vi "Velociprobe_Nanopositioner_Control_RT 3.vi"() -> ()   [LabVIEW 2015] (continued)
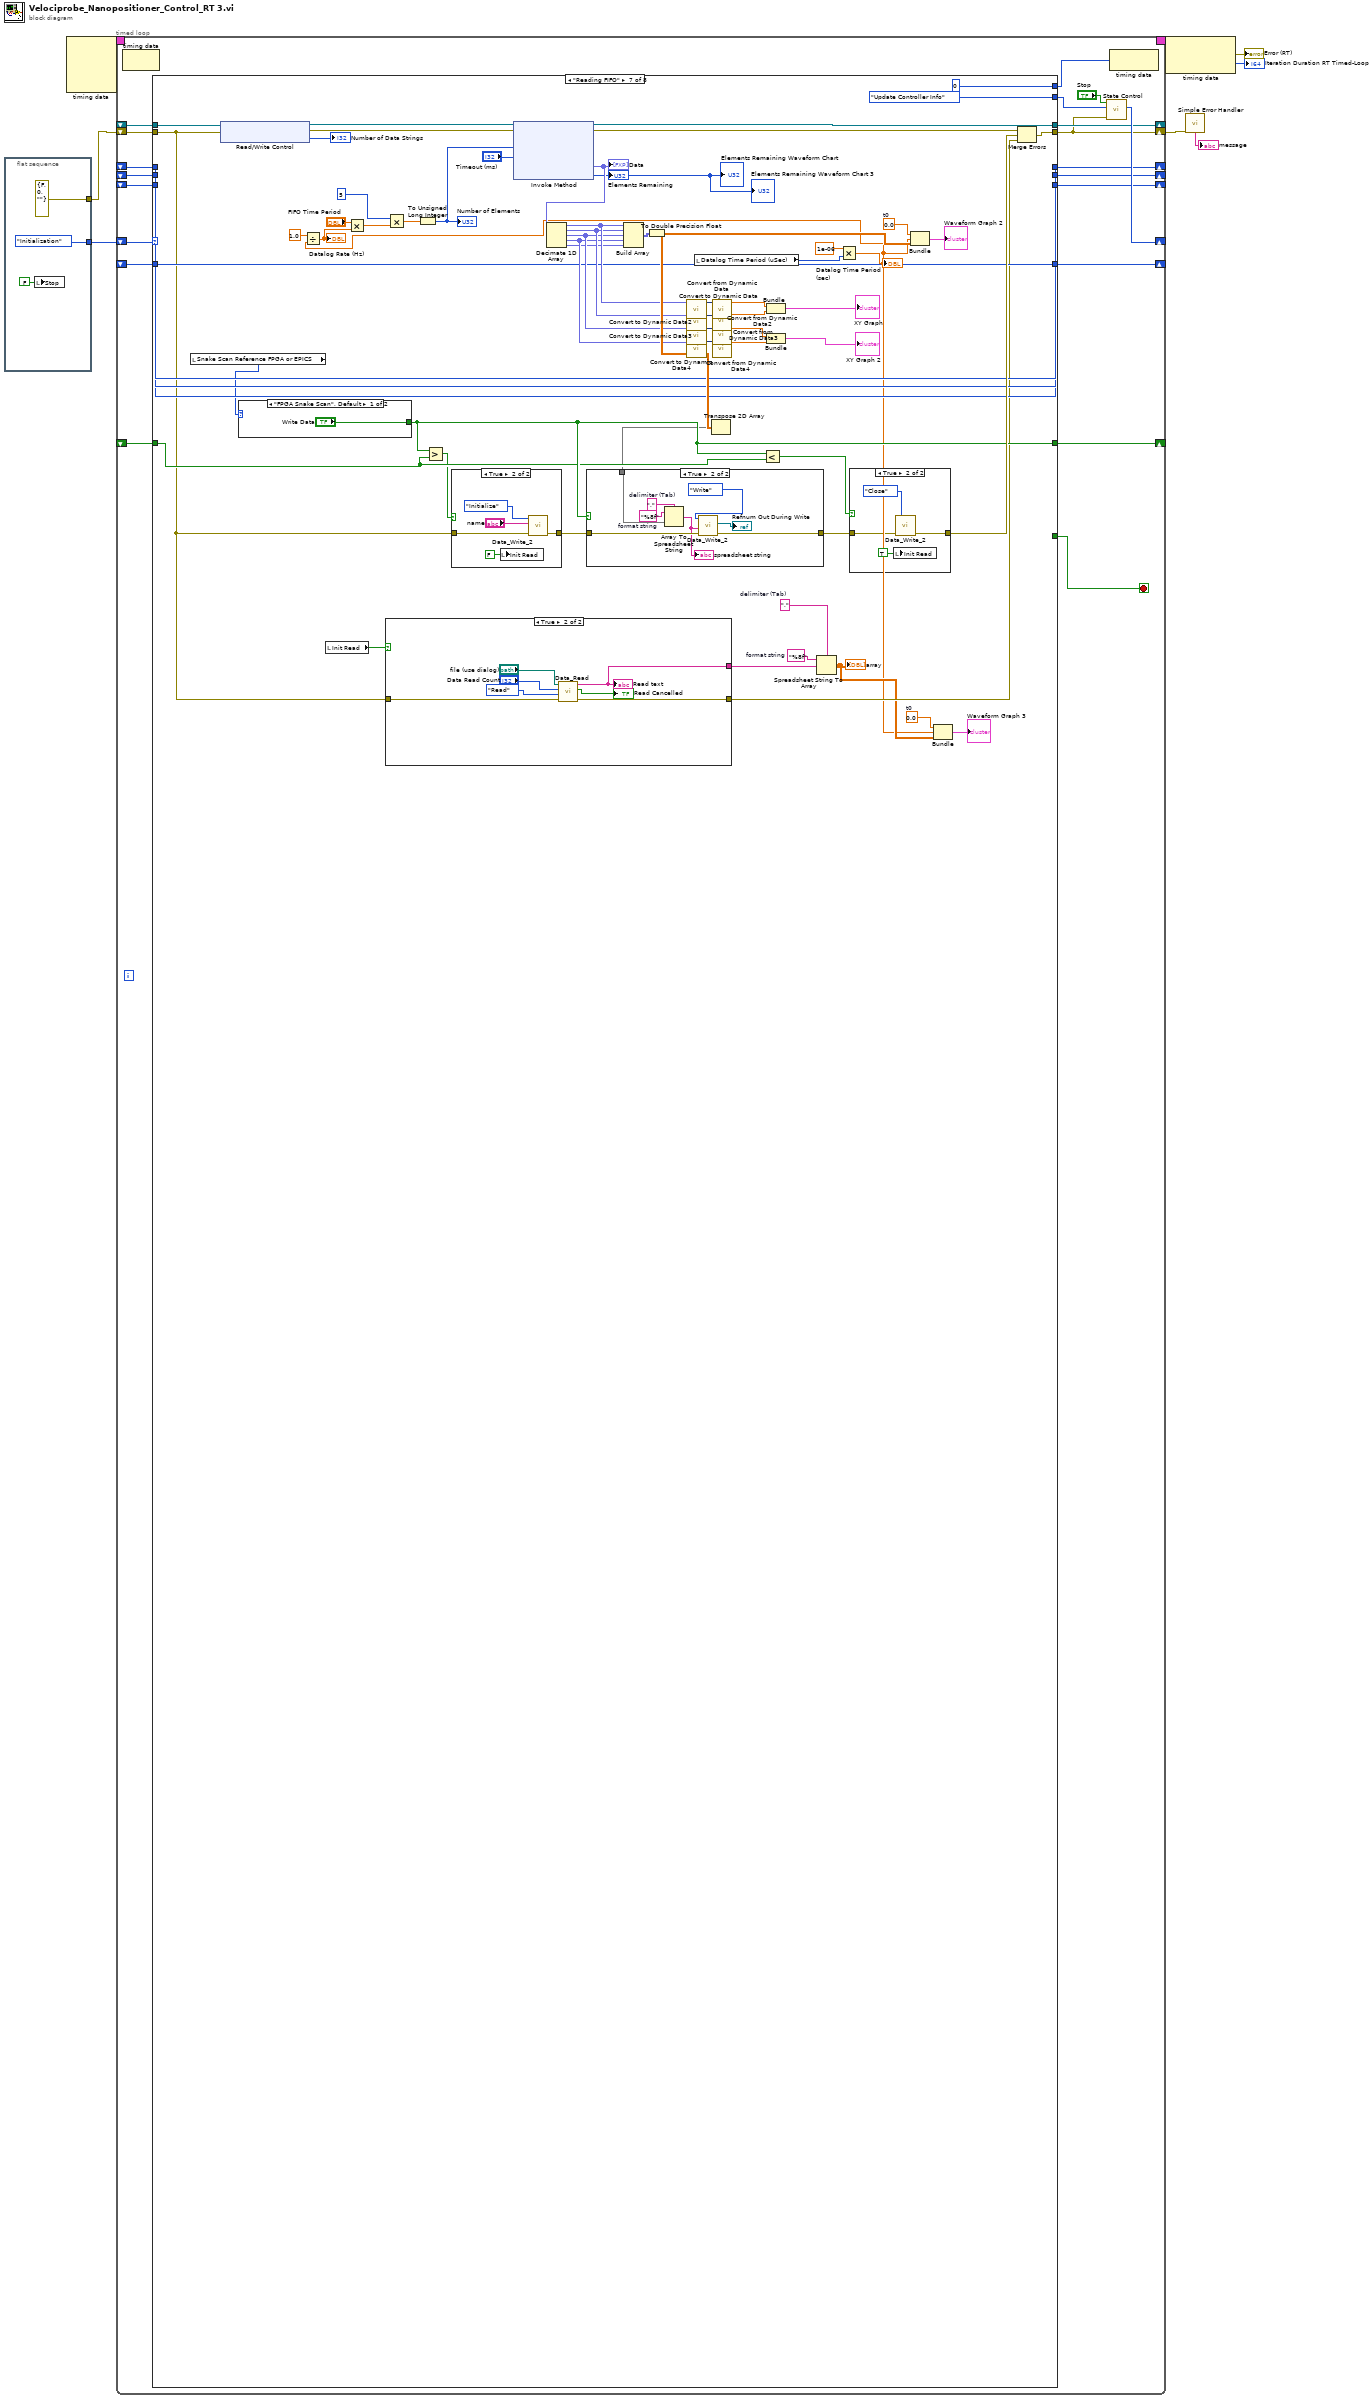
[diagram p0: block diagram]
diagram:
  n1 = flat-sequence {
    tunnel: [State_Enum."Initialization" ("States")] -> w6
    tunnel: [errorcluster {"status"=FALSE, "code"=0, "source"=""} ("error constant")] -> w2
    frame #0 {
      n2 = local write "Stop"(FALSE ("Stop")) -> ()
    }
  }
  n3 = node-c288() -> (w8:T8)  [unwired: 4 in]
  n4 = timed-loop {
    timing: w8 -> [_]
    timing-out: [_] -> w7
    shift-right: [w30] -> _
    shift-left: _ -> [w29]
    shift-right: [w24] -> _
    shift-left: w6 -> [w28]
    shift-right: [w23] -> _
    shift-left: _ -> [w22]
    shift-right: [w21] -> _
    shift-left: _ -> [w20]
    shift-right: [w18] -> _
    shift-left: _ -> [w19]
    shift-right: [w17] -> _
    shift-left: _ -> [w16]
    shift-right: [w15] -> _
    shift-left: _ -> [w12]
    shift-right: [w14] -> w1
    shift-left: w2 -> [w13]
    stop <- w27 stop-if-true
    n5 = node-c288() -> ()  [unwired: 1 in, 1 out]
    n6 = case shown="\"Reading FIFO\"" w28 {
      tunnel: [i64 0 i64 0 i64 0 i64 0 i64 0 i64 0 i64 0 i64 0] -> w31
      tunnel: [w52 w346 w629 w728 w769 w803 w860 w917] -> w30
      tunnel: w29 -> [w52 w346 w629 w728 w769 w803 w859 w917]
      tunnel: [State_Enum."Update Controller Info" State_Enum."Update Reference Info" State_Enum."Update Detector Trigger Info" State_Enum."Update Datalog Info" ("States") State_Enum."Check FPGA Status" State_Enum."Reading FIFO" State_Enum."Update Controller Info" State_Enum."Initialization"] -> w25
      tunnel: [_ _ _ _ _ _ _ w918] -> w27
      tunnel: [w50 w75 w585 w723 w750 w802 w850 w916] -> w23
      tunnel: w22 -> [w50 w75 w584 w723 w750 w802 w850 w916]
      tunnel: [w49 w74 w581 w722 w749 w801 w849 w915] -> w21
      tunnel: w20 -> [w49 w74 w579 w722 w749 w801 w849 w915]
      tunnel: w19 -> [w48 w73 w576 w721 w748 w800 w848 w914]
      tunnel: [w48 w73 w580 w721 w748 w800 w848 w914] -> w18
      tunnel: [w47 w72 w571 w704 w747 w799 w833 w913] -> w17
      tunnel: w16 -> [w47 w72 w571 w703 w747 w799 w833 w913]
      tunnel: [w36 w67 w531 w695 w741 w796 w828 w908] -> w15
      tunnel: [w34 w66 w532 w694 w742 w794 w826 w906] -> w14
      tunnel: w13 -> [w33 w71 w535 w698 w745 w797 w823 w911]
      tunnel: w12 -> [_ w70 w536 w699 w746 w798 w831 w912]
      frame "Initialization", Default {
        w55 = 0  # IRQ Number(s)
        n7 = xnode "Open FPGA VI Reference"("error in"=w33, "resource name"=tag "rio://169.254.76.54/RIO0") -> ("FPGA VI Reference Out"=w45:refnum<k20>, "error out"=w46:errorcluster)
        n8 = xnode "Invoke Method"("FPGA VI Reference In"=w45, "error in"=w46, "Requested Depth"="Requested Depth") -> ("FPGA VI Reference Out"=w44:refnum<k20>, "error out"=w43:errorcluster, "Actual Depth"=→"Actual Depth":u32)
        n9 = xnode "Read/Write Control"("FPGA VI Reference In"=w44, "error in"=w43, "Datalog Time Period (uSec)"="Datalog Time Period (uSec)", "Datalog Cases"="Datalog Cases", "Interrupt Boolean"=FALSE) -> ("FPGA VI Reference Out"=w42:refnum<k20>, "error out"=w41:errorcluster)
        n10 = xnode "Invoke Method"("FPGA VI Reference In"=w42, "error in"=w41, "IRQ Number(s)"=w55, "Timeout (ms)"="IRQ Timeout (ms)") -> ("FPGA VI Reference Out"=w40:refnum<k20>, "error out"=w39:errorcluster, "Timed Out"=→"IRQ Timed Out":bool, "IRQ(s) Asserted"=w57:i32)
        n11 = xnode "Invoke Method"("FPGA VI Reference In"=w40, "error in"=w39, "IRQ Number(s)"=w57) -> ("FPGA VI Reference Out"=w38:refnum<k20>, "error out"=w37:errorcluster)
        n12 = xnode "Read/Write Control"("FPGA VI Reference In"=w38, "error in"=w37) -> ("FPGA VI Reference Out"=w36:refnum<k20>, "error out"=w35:errorcluster, "error out (FPGA)"=w58:errorcluster)
        n13 = invoke on="Waveform Graph 2" class="WFGraph (strict)" method="Reinit To Default"() -> (error out=w51:errorcluster)  [unwired: 3 in, 2 out]
        n14 = Merge Errors "Merge Errors"(w35, w58, w51) -> (w34:errorcluster)
        "Init Read" <- FALSE ("Init Read")
      }
      frame "Update Controller Info" {
        w295 = dbl[] [1.0, 2.0, 4.0, 5.0]  # Index_soscoeff_zz1
        w134 = dbl[] [1.0, 2.0, 4.0, 5.0]  # Index_soscoeff_yz1
        w155 = dbl[] [1.0, 2.0, 4.0, 5.0]  # Index_soscoeff_xz1
        w186 = dbl[] [1.0, 2.0, 4.0, 5.0]  # Index_soscoeff_zy1
        w316 = dbl[] [1.0, 2.0, 4.0, 5.0]  # Index_soscoeff_yy1
        w207 = dbl[] [1.0, 2.0, 4.0, 5.0]  # Index_soscoeff_xy1
        w233 = dbl[] [1.0, 2.0, 4.0, 5.0]  # Index_soscoeff_zx1
        w342 = dbl[] [1.0, 2.0, 4.0, 5.0]  # Index_soscoeff_xx1
        w259 = dbl[] [1.0, 2.0, 4.0, 5.0]  # Index_soscoeff_yx1
        w115 = "%.10f"  # format (%.3f)
        w123 = "%.10f"  # format (%.3f)
        w136 = "%.10f"  # format (%.3f)
        w144 = "%.10f"  # format (%.3f)
        w167 = "%.10f"  # format (%.3f)
        w175 = "%.10f"  # format (%.3f)
        w188 = "%.10f"  # format (%.3f)
        w196 = "%.10f"  # format (%.3f)
        w214 = "%.10f"  # format (%.3f)
        w222 = "%.10f"  # format (%.3f)
        w240 = "%.10f"  # format (%.3f)
        w248 = "%.10f"  # format (%.3f)
        w276 = "%.10f"  # format (%.3f)
        w284 = "%.10f"  # format (%.3f)
        w297 = "%.10f"  # format (%.3f)
        w305 = "%.10f"  # format (%.3f)
        w106 = fxp<+/-,42,9> 0.0 ("fixed-point type")
        w318 = "%.10f"  # format (%.3f)
        w105 = fxp<+/-,64,9> 0.0 ("fixed-point type")
        w331 = "%.10f"  # format (%.3f)
        w350 = 40000000.0  # FPGA Clock Rate (Hz)
        w82 = 1
        n15 = local read "sos gain SF Controller yy1c"() -> (w270:fxp<+/-,42,9>)
        n16 = local read "sos gain SF Controller yz1c"() -> (w91:fxp<+/-,42,9>)
        n17 = local read "sos gain SF Controller yx1c"() -> (w237:fxp<+/-,42,9>)
        n18 = local read "sos gain SF Controller xy1c"() -> (w160:fxp<+/-,42,9>)
        n19 = local read "sos gain SF Controller zy1c"() -> (w165:fxp<+/-,42,9>)
        n20 = local read "sos gain SF Controller xz1c"() -> (w107:fxp<+/-,42,9>)
        n21 = local read "sos gain SF Controller xx1c"() -> (w320:fxp<+/-,42,9>)
        n22 = local read "sos gain SF Controller zz1c"() -> (w268:fxp<+/-,42,9>)
        n23 = local read "sos gain SF Controller zx1c"() -> (w212:fxp<+/-,42,9>)
        n24 = local read "-a01(2) yy1c"() -> (w274:fxp<+/-,64,9>[])
        n25 = local read "-a02(2) yy1c"() -> (w273:fxp<+/-,64,9>[])
        n26 = local read "-a01(2) yz1c"() -> (w112:fxp<+/-,64,9>[])
        n27 = local read "-a02(2) yz1c"() -> (w113:fxp<+/-,64,9>[])
        n28 = local read "-a01(2) yx1c"() -> (w238:fxp<+/-,64,9>[])
        n29 = local read "-a02(2) yx1c"() -> (w234:fxp<+/-,64,9>[])
        n30 = local read "-a01(2) xy1c"() -> (w156:fxp<+/-,64,9>[])
        n31 = local read "-a02(2) xy1c"() -> (w157:fxp<+/-,64,9>[])
        n32 = local read "-a01(2) zy1c"() -> (w161:fxp<+/-,64,9>[])
        n33 = local read "-a02(2) zy1c"() -> (w162:fxp<+/-,64,9>[])
        n34 = local read "-a01(2) xz1c"() -> (w111:fxp<+/-,64,9>[])
        n35 = local read "-a02(2) xz1c"() -> (w110:fxp<+/-,64,9>[])
        n36 = local read "-a01(2) xx1c"() -> (w329:fxp<+/-,64,9>[])
        n37 = local read "-a02(2) xx1c"() -> (w328:fxp<+/-,64,9>[])
        n38 = local read "-a01(2) zz1c"() -> (w269:fxp<+/-,64,9>[])
        n39 = local read "-a02(2) zz1c"() -> (w265:fxp<+/-,64,9>[])
        n40 = local read "-a01(2) zx1c"() -> (w208:fxp<+/-,64,9>[])
        n41 = local read "-a02(2) zx1c"() -> (w209:fxp<+/-,64,9>[])
        n42 = local read "b01(2) yy1c"() -> (w272:fxp<+/-,64,9>[])
        n43 = local read "b02(2) yy1c"() -> (w271:fxp<+/-,64,9>[])
        n44 = local read "b01(2) yz1c"() -> (w77:fxp<+/-,64,9>[])
        n45 = local read "b02(2) yz1c"() -> (w76:fxp<+/-,64,9>[])
        n46 = local read "b01(2) yx1c"() -> (w235:fxp<+/-,64,9>[])
        n47 = local read "b02(2) yx1c"() -> (w236:fxp<+/-,64,9>[])
        n48 = local read "b01(2) xy1c"() -> (w158:fxp<+/-,64,9>[])
        n49 = local read "b02(2) xy1c"() -> (w159:fxp<+/-,64,9>[])
        n50 = local read "b01(2) zy1c"() -> (w163:fxp<+/-,64,9>[])
        n51 = local read "b02(2) zy1c"() -> (w164:fxp<+/-,64,9>[])
        n52 = local read "b01(2) xz1c"() -> (w109:fxp<+/-,64,9>[])
        n53 = local read "b02(2) xz1c"() -> (w108:fxp<+/-,64,9>[])
        n54 = local read "b01(2) xx1c"() -> (w327:fxp<+/-,64,9>[])
        n55 = local read "b02(2) xx1c"() -> (w326:fxp<+/-,64,9>[])
        n56 = local read "b01(2) zz1c"() -> (w266:fxp<+/-,64,9>[])
        n57 = local read "b02(2) zz1c"() -> (w267:fxp<+/-,64,9>[])
        n58 = local read "b01(2) zx1c"() -> (w210:fxp<+/-,64,9>[])
        n59 = local read "b02(2) zx1c"() -> (w211:fxp<+/-,64,9>[])
        n60 = Or(x="Optics Z Reset", y="Reset All") -> (x .or. y?=w104:bool)
        n61 = Or(x="Sample Z Reset", y="Reset All") -> (x .or. y?=w101:bool)
        n62 = Or(x="Optics X Reset", y="Reset All") -> (x .or. y?=w263:bool)
        n63 = Or(x="Optics Y Reset", y="Reset All") -> (x .or. y?=w261:bool)
        n64 = Or(x="Sample X Reset", y="Reset All") -> (x .or. y?=w103:bool)
        n65 = Or(x="Sample Y Reset", y="Reset All") -> (x .or. y?=w102:bool)
        n66 = call-poly <vilib>:"Read Delimited Spreadsheet.vi"("file path (dialog if empty)"="file path soscoeff_xx1", "format (%.3f)"=w331) -> ("all rows"=w330:dbl[][])  [unwired: 8 in, 5 out]
        n67 = call-poly <vilib>:"Read Delimited Spreadsheet.vi"("file path (dialog if empty)"="file path soscoeff_zy1", "format (%.3f)"=w175) -> ("all rows"=w174:dbl[][])  [unwired: 8 in, 5 out]
        n68 = call-poly <vilib>:"Read Delimited Spreadsheet.vi"("file path (dialog if empty)"="file path soscoeff_xy1", "format (%.3f)"=w196) -> ("all rows"=w195:dbl[][])  [unwired: 8 in, 5 out]
        n69 = call-poly <vilib>:"Read Delimited Spreadsheet.vi"("file path (dialog if empty)"="file path soscoeff_zx1", "format (%.3f)"=w222) -> ("all rows"=w221:dbl[][])  [unwired: 8 in, 5 out]
        n70 = call-poly <vilib>:"Read Delimited Spreadsheet.vi"("file path (dialog if empty)"="file path soscoeff_xz1", "format (%.3f)"=w144) -> ("all rows"=w143:dbl[][])  [unwired: 8 in, 5 out]
        n71 = call-poly <vilib>:"Read Delimited Spreadsheet.vi"("file path (dialog if empty)"="file path soscoeff_yx1", "format (%.3f)"=w248) -> ("all rows"=w247:dbl[][])  [unwired: 8 in, 5 out]
        n72 = call-poly <vilib>:"Read Delimited Spreadsheet.vi"("file path (dialog if empty)"="file path soscoeff_yy1", "format (%.3f)"=w305) -> ("all rows"=w304:dbl[][])  [unwired: 8 in, 5 out]
        n73 = call-poly <vilib>:"Read Delimited Spreadsheet.vi"("file path (dialog if empty)"="file path soscoeff_yz1", "format (%.3f)"=w123) -> ("all rows"=w122:dbl[][])  [unwired: 8 in, 5 out]
        n74 = call-poly <vilib>:"Read Delimited Spreadsheet.vi"("file path (dialog if empty)"="file path soscoeff_zz1", "format (%.3f)"=w284) -> ("all rows"=w283:dbl[][])  [unwired: 8 in, 5 out]
        n75 = Transpose 2D Array(2D array=w330) -> (transposed array=w341:dbl[][])
        n76 = Transpose 2D Array(2D array=w174) -> (transposed array=w185:dbl[][])
        n77 = Transpose 2D Array(2D array=w195) -> (transposed array=w206:dbl[][])
        n78 = Transpose 2D Array(2D array=w221) -> (transposed array=w232:dbl[][])
        n79 = Transpose 2D Array(2D array=w143) -> (transposed array=w154:dbl[][])
        n80 = Transpose 2D Array(2D array=w247) -> (transposed array=w258:dbl[][])
        n81 = Transpose 2D Array(2D array=w304) -> (transposed array=w315:dbl[][])
        n82 = Transpose 2D Array(2D array=w122) -> (transposed array=w133:dbl[][])
        n83 = Transpose 2D Array(2D array=w283) -> (transposed array=w294:dbl[][])
        n84 = call-poly <vilib>:"Read Delimited Spreadsheet.vi"("file path (dialog if empty)"="file path sos gain SF Controller_xx1", "format (%.3f)"=w318) -> ("all rows"=w317:dbl[][])  [unwired: 8 in, 5 out]
        n85 = call-poly <vilib>:"Read Delimited Spreadsheet.vi"("file path (dialog if empty)"="file path sos gain SF Controller_zy1", "format (%.3f)"=w167) -> ("all rows"=w166:dbl[][])  [unwired: 8 in, 5 out]
        n86 = call-poly <vilib>:"Read Delimited Spreadsheet.vi"("file path (dialog if empty)"="file path sos gain SF Controller_xy1", "format (%.3f)"=w188) -> ("all rows"=w187:dbl[][])  [unwired: 8 in, 5 out]
        n87 = call-poly <vilib>:"Read Delimited Spreadsheet.vi"("file path (dialog if empty)"="file path sos gain SF Controller_zx1", "format (%.3f)"=w214) -> ("all rows"=w213:dbl[][])  [unwired: 8 in, 5 out]
        n88 = call-poly <vilib>:"Read Delimited Spreadsheet.vi"("file path (dialog if empty)"="file path sos gain SF Controller_xz1", "format (%.3f)"=w136) -> ("all rows"=w135:dbl[][])  [unwired: 8 in, 5 out]
        n89 = call-poly <vilib>:"Read Delimited Spreadsheet.vi"("file path (dialog if empty)"="file path sos gain SF Controller_yx1", "format (%.3f)"=w240) -> ("all rows"=w239:dbl[][])  [unwired: 8 in, 5 out]
        n90 = call-poly <vilib>:"Read Delimited Spreadsheet.vi"("file path (dialog if empty)"="file path sos gain SF Controller_yy1", "format (%.3f)"=w297) -> ("all rows"=w296:dbl[][])  [unwired: 8 in, 5 out]
        n91 = call-poly <vilib>:"Read Delimited Spreadsheet.vi"("file path (dialog if empty)"="file path sos gain SF Controller_yz1", "format (%.3f)"=w115) -> ("all rows"=w114:dbl[][])  [unwired: 8 in, 5 out]
        n92 = call-poly <vilib>:"Read Delimited Spreadsheet.vi"("file path (dialog if empty)"="file path sos gain SF Controller_zz1", "format (%.3f)"=w276) -> ("all rows"=w275:dbl[][])  [unwired: 8 in, 5 out]
        n93 = xnode "Read/Write Control"("FPGA VI Reference In"=w70, "error in"=w71, "Controller Time Period (uSec)"="Controller Time Period (uSec)", "Controller Output Time Period (uSec)"="Controller Output Time Period (uSec)", "System Loop Type"="System Loop Type", "Controller Output Upper Limit"="Controller Output Upper Limit", "Controller Output Lower Limit"="Controller Output Lower Limit", "X-Stage nm to V Scaling"="X-Stage nm to V Scaling", "X-Stage Scaling Direction"="X-Stage Scaling Direction", "Y-Stage nm to V Scaling"="Y-Stage nm to V Scaling", "Z-Stage nm to V Scaling"="Z-Stage nm to V Scaling", "Plant Output Time Period (uSec)"="Plant Output Time Period (uSec)", "Reset Optics X"=w263, "Reset Optics Y"=w261, "Reset Optics Z"=w104, "Reset Sample X"=w103, "Reset Sample Y"=w102, "Reset Sample Z"=w101, "Optics X Stage Resolution (nm)"="Optics X Stage Resolution (nm)", "Optics Y Stage Resolution (nm)"="Optics Y Stage Resolution (nm)", "Optics Z Stage Resolution (nm)"="Optics Z Stage Resolution (nm)", "Sample X Stage Resolution (nm)"="Sample X Stage Resolution (nm)", "Sample Y Stage Resolution (nm)"="Sample Y Stage Resolution (nm)", "Sample Z Stage Resolution (nm)"="Sample Z Stage Resolution (nm)", "Scaling mV to V"="Scaling mV to V", "-a01(2) xx1"=w329, "-a02(2) xx1"=w328, "b01(2) xx1"=w327, "b02(2) xx1"=w326, "sos gain SF Controller xx1"=w320, "-a01(2) yy1"=w274, "-a02(2) yy1"=w273, "b01(2) yy1"=w272, "b02(2) yy1"=w271, "sos gain SF Controller yy1"=w270, "-a01(2) zz1"=w269, "-a02(2) zz1"=w265, "b01(2) zz1"=w266, "b02(2) zz1"=w267, "sos gain SF Controller zz1"=w268, "-a01(2) yx1"=w238, "-a02(2) yx1"=w234, "b01(2) yx1"=w235, "b02(2) yx1"=w236, "sos gain SF Controller yx1"=w237, "-a01(2) zx1"=w208, "-a02(2) zx1"=w209, "b01(2) zx1"=w210, "b02(2) zx1"=w211, "sos gain SF Controller zx1"=w212, "-a01(2) xy1"=w156, "-a02(2) xy1"=w157, "b01(2) xy1"=w158, "b02(2) xy1"=w159, "sos gain SF Controller xy1"=w160, "-a01(2) zy1"=w161, "-a02(2) zy1"=w162, "b01(2) zy1"=w163, "b02(2) zy1"=w164, "sos gain SF Controller zy1"=w165, "-a01(2) xz1"=w111, "-a02(2) xz1"=w110, "b01(2) xz1"=w109, "b02(2) xz1"=w108, "sos gain SF Controller xz1"=w107, "-a01(2) yz1"=w112, "-a02(2) yz1"=w113, "b01(2) yz1"=w77, "b02(2) yz1"=w76, "sos gain SF Controller yz1"=w91, "Analog Input Time Period (uSec)"="Analog Input Time Period (uSec)", "Optics and or Sample Stage"="Optics and or Sample Stage", "Y-Stage Scaling Direction"="Y-Stage Scaling Direction", "Z-Stage Scaling Direction"="Z-Stage Scaling Direction") -> ("FPGA VI Reference Out"=w69:refnum<k20>, "error out"=w68:errorcluster)
        n94 = for {
          tunnel: w342 -> [w519] mode=indexing
          tunnel: w341 -> [w518]
          tunnel: [w517] -> _ mode=indexing
          shift-right: [w517] -> w333
          shift-left: _ -> [w516]
          shift-left: _ -> [w515]
          shift-left: _ -> [w514]
          tunnel: [w516] -> w334
          tunnel: [w515] -> w335
          tunnel: [w514] -> w336
          n95 = Index Array "Index Array"(array=w518, index (row)=w519) -> (element=w517:dbl[])  [unwired: 1 in]
        }
        n96 = Index Array(array=w317, index (row)=0 ("index (row) 6")) -> (element=w325:dbl[])  [unwired: 1 in]
        n97 = for {
          tunnel: w186 -> [w417] mode=indexing
          tunnel: w185 -> [w416]
          tunnel: [w415] -> _ mode=indexing
          shift-right: [w415] -> w177
          shift-left: _ -> [w414]
          shift-left: _ -> [w413]
          shift-left: _ -> [w412]
          tunnel: [w414] -> w178
          tunnel: [w413] -> w179
          tunnel: [w412] -> w180
          n98 = Index Array "Index Array"(array=w416, index (row)=w417) -> (element=w415:dbl[])  [unwired: 1 in]
        }
        n99 = Index Array(array=w166, index (row)=0 ("index (row) 18")) -> (element=w173:dbl[])  [unwired: 1 in]
        n100 = for {
          tunnel: w207 -> [w434] mode=indexing
          tunnel: w206 -> [w433]
          tunnel: [w432] -> _ mode=indexing
          shift-right: [w432] -> w198
          shift-left: _ -> [w431]
          shift-left: _ -> [w430]
          shift-left: _ -> [w429]
          tunnel: [w431] -> w199
          tunnel: [w430] -> w200
          tunnel: [w429] -> w201
          n101 = Index Array "Index Array"(array=w433, index (row)=w434) -> (element=w432:dbl[])  [unwired: 1 in]
        }
        n102 = Index Array(array=w187, index (row)=0 ("index (row) 16")) -> (element=w194:dbl[])  [unwired: 1 in]
        n103 = for {
          tunnel: w233 -> [w451] mode=indexing
          tunnel: w232 -> [w450]
          tunnel: [w449] -> _ mode=indexing
          shift-right: [w449] -> w224
          shift-left: _ -> [w448]
          shift-left: _ -> [w447]
          shift-left: _ -> [w446]
          tunnel: [w448] -> w225
          tunnel: [w447] -> w226
          tunnel: [w446] -> w227
          n104 = Index Array "Index Array"(array=w450, index (row)=w451) -> (element=w449:dbl[])  [unwired: 1 in]
        }
        n105 = Index Array(array=w213, index (row)=0 ("index (row) 14")) -> (element=w220:dbl[])  [unwired: 1 in]
        n106 = for {
          tunnel: w155 -> [w400] mode=indexing
          tunnel: w154 -> [w399]
          tunnel: [w398] -> _ mode=indexing
          shift-right: [w398] -> w146
          shift-left: _ -> [w397]
          shift-left: _ -> [w396]
          shift-left: _ -> [w395]
          tunnel: [w397] -> w147
          tunnel: [w396] -> w148
          tunnel: [w395] -> w149
          n107 = Index Array "Index Array"(array=w399, index (row)=w400) -> (element=w398:dbl[])  [unwired: 1 in]
        }
        n108 = Index Array(array=w135, index (row)=0 ("index (row) 20")) -> (element=w142:dbl[])  [unwired: 1 in]
        n109 = for {
          tunnel: w259 -> [w468] mode=indexing
          tunnel: w258 -> [w467]
          tunnel: [w466] -> _ mode=indexing
          shift-right: [w466] -> w250
          shift-left: _ -> [w465]
          shift-left: _ -> [w464]
          shift-left: _ -> [w463]
          tunnel: [w465] -> w251
          tunnel: [w464] -> w252
          tunnel: [w463] -> w253
          n110 = Index Array "Index Array"(array=w467, index (row)=w468) -> (element=w466:dbl[])  [unwired: 1 in]
        }
        n111 = Index Array(array=w239, index (row)=0 ("index (row) 12")) -> (element=w246:dbl[])  [unwired: 1 in]
        n112 = for {
          tunnel: w316 -> [w502] mode=indexing
          tunnel: w315 -> [w501]
          tunnel: [w500] -> _ mode=indexing
          shift-right: [w500] -> w307
          shift-left: _ -> [w499]
          shift-left: _ -> [w498]
          shift-left: _ -> [w497]
          tunnel: [w499] -> w308
          tunnel: [w498] -> w309
          tunnel: [w497] -> w310
          n113 = Index Array "Index Array"(array=w501, index (row)=w502) -> (element=w500:dbl[])  [unwired: 1 in]
        }
        n114 = Index Array(array=w296, index (row)=0 ("index (row) 8")) -> (element=w303:dbl[])  [unwired: 1 in]
        n115 = for {
          tunnel: w134 -> [w383] mode=indexing
          tunnel: w133 -> [w382]
          tunnel: [w381] -> _ mode=indexing
          shift-right: [w381] -> w125
          shift-left: _ -> [w380]
          shift-left: _ -> [w379]
          shift-left: _ -> [w378]
          tunnel: [w380] -> w126
          tunnel: [w379] -> w127
          tunnel: [w378] -> w128
          n116 = Index Array "Index Array"(array=w382, index (row)=w383) -> (element=w381:dbl[])  [unwired: 1 in]
        }
        n117 = Index Array(array=w114, index (row)=0 ("index (row) 22")) -> (element=w121:dbl[])  [unwired: 1 in]
        n118 = Index Array(array=w275, index (row)=0 ("index (row) 10")) -> (element=w282:dbl[])  [unwired: 1 in]
        n119 = for {
          tunnel: w295 -> [w485] mode=indexing
          tunnel: w294 -> [w484]
          tunnel: [w483] -> _ mode=indexing
          shift-right: [w483] -> w286
          shift-left: _ -> [w482]
          shift-left: _ -> [w481]
          shift-left: _ -> [w480]
          tunnel: [w482] -> w287
          tunnel: [w481] -> w288
          tunnel: [w480] -> w289
          n120 = Index Array "Index Array"(array=w484, index (row)=w485) -> (element=w483:dbl[])  [unwired: 1 in]
        }
        n121 = Index Array(array=w325, index=0 ("index (row) 7")) -> (element=w323:dbl)
        n122 = Index Array(array=w173, index=0 ("index (row) 19")) -> (element=w171:dbl)
        n123 = Index Array(array=w194, index=0 ("index (row) 17")) -> (element=w192:dbl)
        n124 = Index Array(array=w220, index=0 ("index (row) 15")) -> (element=w218:dbl)
        n125 = Index Array(array=w142, index=0 ("index (row) 21")) -> (element=w140:dbl)
        n126 = Index Array(array=w246, index=0 ("index (row) 13")) -> (element=w244:dbl)
        n127 = Index Array(array=w303, index=0 ("index (row) 9")) -> (element=w301:dbl)
        n128 = Index Array(array=w121, index=0 ("index (row) 23")) -> (element=w119:dbl)
        n129 = Index Array(array=w282, index=0 ("index (row) 11")) -> (element=w280:dbl)
        n130 = xnode "Read/Write Control"("FPGA VI Reference In"=w69, "error in"=w68) -> ("FPGA VI Reference Out"=w67:refnum<k20>, "error out"=w66:errorcluster, "PI X-Stage Input (V)"=→"PI X-Stage Input (V)":fxp<+/-,20,5>, "PI Y-Stage Input (V)"=→"PI Y-Stage Input (V)":fxp<+/-,20,5>, "PI Z-Stage Input (V)"=→"PI Z-Stage Input (V)":fxp<+/-,20,5>, "X-Stage Input In Range?"=→"X-Stage Input In Range?":bool, "Y-Stage Input In Range?"=→"Y-Stage Input In Range?":bool, "Z-Stage Input In Range?"=→"Z-Stage Input In Range?":bool, "Measured Controller Time Period (Ticks)"=w351:u32, "Measured Controller Output Time Period (Ticks)"=w348:u32, "Measured Plant Output Time Period (Ticks)"=w83:u32, "Measured Analog Input Time Period (Ticks)"=→"Measured Analog Input Time Period (Ticks)":u32)
        "Measured Controller Time Period (Ticks)" <- w351
        "Measured Controller Output Time Period (Ticks)" <- w348
        "Measured Plant Output Time Period (Ticks)" <- w83
        n131 = To Fixed-Point(fixed-point type=w106, number=w192) -> (fixed-point=→"sos gain SF Controller xy1c":fxp<+/-,42,9>)
        n132 = To Fixed-Point(fixed-point type=w106, number=w301) -> (fixed-point=→"sos gain SF Controller yy1c":fxp<+/-,42,9>)
        n133 = To Fixed-Point(fixed-point type=w106, number=w171) -> (fixed-point=→"sos gain SF Controller zy1c":fxp<+/-,42,9>)
        n134 = To Fixed-Point(fixed-point type=w106, number=w140) -> (fixed-point=→"sos gain SF Controller xz1c":fxp<+/-,42,9>)
        n135 = To Fixed-Point(fixed-point type=w106, number=w119) -> (fixed-point=→"sos gain SF Controller yz1c":fxp<+/-,42,9>)
        n136 = To Fixed-Point(fixed-point type=w106, number=w244) -> (fixed-point=→"sos gain SF Controller yx1c":fxp<+/-,42,9>)
        n137 = To Fixed-Point(fixed-point type=w106, number=w218) -> (fixed-point=→"sos gain SF Controller zx1c":fxp<+/-,42,9>)
        n138 = To Fixed-Point(fixed-point type=w106, number=w280) -> (fixed-point=→"sos gain SF Controller zz1c":fxp<+/-,42,9>)
        n139 = To Fixed-Point(fixed-point type=w106, number=w323) -> (fixed-point=→"sos gain SF Controller xx1c":fxp<+/-,42,9>)
        n140 = Divide(x=w82, y=w350) -> (x/y=w84:dbl)
        n141 = Multiply(x=w84, y=w351) -> (x*y=w352:dbl)
        "Measured Controller Loop Rate (secs)" <- w352
        n142 = Multiply(x=w84, y=w348) -> (x*y=w360:dbl)
        "Measured Controller Output Loop Rate (secs)" <- w360
        n143 = Multiply(x=w84, y=w83) -> (x*y=w356:dbl)
        "Measured Plant Output Loop Rate (secs)" <- w356
        n144 = Multiply(x=w84, y=w83) -> (x*y=w88:dbl)
        "Measured Analog Input Loop Rate (secs)" <- w88
        n145 = Divide(x=w82, y=w352) -> (x/y=w363:dbl)
        n146 = Divide(x=w82, y=w360) -> (x/y=w359:dbl)
        n147 = Divide(x=w82, y=w356) -> (x/y=w355:dbl)
        n148 = Divide(x=w82, y=w88) -> (x/y=w87:dbl)
        n149 = for {
          tunnel: w178 -> [w428] mode=indexing
          tunnel: [w427] -> w184 mode=indexing
          tunnel: w177 -> [w426] mode=indexing
          tunnel: w180 -> [w425] mode=indexing
          tunnel: w179 -> [w424] mode=indexing
          tunnel: [w423] -> w183 mode=indexing
          tunnel: [w422] -> w182 mode=indexing
          tunnel: [w421] -> w181 mode=indexing
          tunnel: w105 -> [w418]
          n150 = Negate(x=w428) -> (-x=w420:dbl)
          n151 = Negate(x=w426) -> (-x=w419:dbl)
          n152 = To Fixed-Point(fixed-point type=w418, number=w420) -> (fixed-point=w427:fxp<+/-,64,9>)
          n153 = To Fixed-Point(fixed-point type=w418, number=w419) -> (fixed-point=w423:fxp<+/-,64,9>)
          n154 = To Fixed-Point(fixed-point type=w418, number=w425) -> (fixed-point=w422:fxp<+/-,64,9>)
          n155 = To Fixed-Point(fixed-point type=w418, number=w424) -> (fixed-point=w421:fxp<+/-,64,9>)
        }
        "-a01(2) zy1c" <- w184
        "-a02(2) zy1c" <- w183
        "b01(2) zy1c" <- w182
        "b02(2) zy1c" <- w181
        n156 = for {
          tunnel: w334 -> [w530] mode=indexing
          tunnel: [w529] -> w340 mode=indexing
          tunnel: w333 -> [w528] mode=indexing
          tunnel: w336 -> [w527] mode=indexing
          tunnel: w335 -> [w526] mode=indexing
          tunnel: [w525] -> w339 mode=indexing
          tunnel: [w524] -> w338 mode=indexing
          tunnel: [w523] -> w337 mode=indexing
          tunnel: w105 -> [w520]
          n157 = Negate(x=w530) -> (-x=w522:dbl)
          n158 = Negate(x=w528) -> (-x=w521:dbl)
          n159 = To Fixed-Point(fixed-point type=w520, number=w522) -> (fixed-point=w529:fxp<+/-,64,9>)
          n160 = To Fixed-Point(fixed-point type=w520, number=w521) -> (fixed-point=w525:fxp<+/-,64,9>)
          n161 = To Fixed-Point(fixed-point type=w520, number=w527) -> (fixed-point=w524:fxp<+/-,64,9>)
          n162 = To Fixed-Point(fixed-point type=w520, number=w526) -> (fixed-point=w523:fxp<+/-,64,9>)
        }
        "-a01(2) xx1c" <- w340
        "-a02(2) xx1c" <- w339
        "b01(2) xx1c" <- w338
        "b02(2) xx1c" <- w337
        n163 = for {
          tunnel: w199 -> [w445] mode=indexing
          tunnel: [w444] -> w205 mode=indexing
          tunnel: w198 -> [w443] mode=indexing
          tunnel: w201 -> [w442] mode=indexing
          tunnel: w200 -> [w441] mode=indexing
          tunnel: [w440] -> w204 mode=indexing
          tunnel: [w439] -> w203 mode=indexing
          tunnel: [w438] -> w202 mode=indexing
          tunnel: w105 -> [w435]
          n164 = Negate(x=w445) -> (-x=w437:dbl)
          n165 = Negate(x=w443) -> (-x=w436:dbl)
          n166 = To Fixed-Point(fixed-point type=w435, number=w437) -> (fixed-point=w444:fxp<+/-,64,9>)
          n167 = To Fixed-Point(fixed-point type=w435, number=w436) -> (fixed-point=w440:fxp<+/-,64,9>)
          n168 = To Fixed-Point(fixed-point type=w435, number=w442) -> (fixed-point=w439:fxp<+/-,64,9>)
          n169 = To Fixed-Point(fixed-point type=w435, number=w441) -> (fixed-point=w438:fxp<+/-,64,9>)
        }
        "-a01(2) xy1c" <- w205
        "-a02(2) xy1c" <- w204
        "b01(2) xy1c" <- w203
        "b02(2) xy1c" <- w202
        n170 = for {
          tunnel: w147 -> [w411] mode=indexing
          tunnel: [w410] -> w153 mode=indexing
          tunnel: w146 -> [w409] mode=indexing
          tunnel: w149 -> [w408] mode=indexing
          tunnel: w148 -> [w407] mode=indexing
          tunnel: [w406] -> w152 mode=indexing
          tunnel: [w405] -> w151 mode=indexing
          tunnel: [w404] -> w150 mode=indexing
          tunnel: w105 -> [w401]
          n171 = Negate(x=w411) -> (-x=w403:dbl)
          n172 = Negate(x=w409) -> (-x=w402:dbl)
          n173 = To Fixed-Point(fixed-point type=w401, number=w403) -> (fixed-point=w410:fxp<+/-,64,9>)
          n174 = To Fixed-Point(fixed-point type=w401, number=w402) -> (fixed-point=w406:fxp<+/-,64,9>)
          n175 = To Fixed-Point(fixed-point type=w401, number=w408) -> (fixed-point=w405:fxp<+/-,64,9>)
          n176 = To Fixed-Point(fixed-point type=w401, number=w407) -> (fixed-point=w404:fxp<+/-,64,9>)
        }
        "-a01(2) xz1c" <- w153
        "-a02(2) xz1c" <- w152
        "b01(2) xz1c" <- w151
        "b02(2) xz1c" <- w150
        n177 = for {
          tunnel: w308 -> [w513] mode=indexing
          tunnel: [w512] -> w314 mode=indexing
          tunnel: w307 -> [w511] mode=indexing
          tunnel: w310 -> [w510] mode=indexing
          tunnel: w309 -> [w509] mode=indexing
          tunnel: [w508] -> w313 mode=indexing
          tunnel: [w507] -> w312 mode=indexing
          tunnel: [w506] -> w311 mode=indexing
          tunnel: w105 -> [w503]
          n178 = Negate(x=w513) -> (-x=w505:dbl)
          n179 = Negate(x=w511) -> (-x=w504:dbl)
          n180 = To Fixed-Point(fixed-point type=w503, number=w505) -> (fixed-point=w512:fxp<+/-,64,9>)
          n181 = To Fixed-Point(fixed-point type=w503, number=w504) -> (fixed-point=w508:fxp<+/-,64,9>)
          n182 = To Fixed-Point(fixed-point type=w503, number=w510) -> (fixed-point=w507:fxp<+/-,64,9>)
          n183 = To Fixed-Point(fixed-point type=w503, number=w509) -> (fixed-point=w506:fxp<+/-,64,9>)
        }
        "-a01(2) yy1c" <- w314
        "-a02(2) yy1c" <- w313
        "b01(2) yy1c" <- w312
        "b02(2) yy1c" <- w311
        n184 = for {
          tunnel: w225 -> [w462] mode=indexing
          tunnel: [w461] -> w231 mode=indexing
          tunnel: w224 -> [w460] mode=indexing
          tunnel: w227 -> [w459] mode=indexing
          tunnel: w226 -> [w458] mode=indexing
          tunnel: [w457] -> w230 mode=indexing
          tunnel: [w456] -> w229 mode=indexing
          tunnel: [w455] -> w228 mode=indexing
          tunnel: w105 -> [w452]
          n185 = Negate(x=w462) -> (-x=w454:dbl)
          n186 = Negate(x=w460) -> (-x=w453:dbl)
          n187 = To Fixed-Point(fixed-point type=w452, number=w454) -> (fixed-point=w461:fxp<+/-,64,9>)
          n188 = To Fixed-Point(fixed-point type=w452, number=w453) -> (fixed-point=w457:fxp<+/-,64,9>)
          n189 = To Fixed-Point(fixed-point type=w452, number=w459) -> (fixed-point=w456:fxp<+/-,64,9>)
          n190 = To Fixed-Point(fixed-point type=w452, number=w458) -> (fixed-point=w455:fxp<+/-,64,9>)
        }
        "-a01(2) zx1c" <- w231
        "-a02(2) zx1c" <- w230
        "b01(2) zx1c" <- w229
        "b02(2) zx1c" <- w228
        n191 = for {
          tunnel: w251 -> [w479] mode=indexing
          tunnel: [w478] -> w257 mode=indexing
          tunnel: w250 -> [w477] mode=indexing
          tunnel: w253 -> [w476] mode=indexing
          tunnel: w252 -> [w475] mode=indexing
          tunnel: [w474] -> w256 mode=indexing
          tunnel: [w473] -> w255 mode=indexing
          tunnel: [w472] -> w254 mode=indexing
          tunnel: w105 -> [w469]
          n192 = Negate(x=w479) -> (-x=w471:dbl)
          n193 = Negate(x=w477) -> (-x=w470:dbl)
          n194 = To Fixed-Point(fixed-point type=w469, number=w471) -> (fixed-point=w478:fxp<+/-,64,9>)
          n195 = To Fixed-Point(fixed-point type=w469, number=w470) -> (fixed-point=w474:fxp<+/-,64,9>)
          n196 = To Fixed-Point(fixed-point type=w469, number=w476) -> (fixed-point=w473:fxp<+/-,64,9>)
          n197 = To Fixed-Point(fixed-point type=w469, number=w475) -> (fixed-point=w472:fxp<+/-,64,9>)
        }
        "-a01(2) yx1c" <- w257
        "-a02(2) yx1c" <- w256
        "b01(2) yx1c" <- w255
        "b02(2) yx1c" <- w254
        n198 = for {
          tunnel: w126 -> [w394] mode=indexing
          tunnel: [w393] -> w132 mode=indexing
          tunnel: w125 -> [w392] mode=indexing
          tunnel: w128 -> [w391] mode=indexing
          tunnel: w127 -> [w390] mode=indexing
          tunnel: [w389] -> w131 mode=indexing
          tunnel: [w388] -> w130 mode=indexing
          tunnel: [w387] -> w129 mode=indexing
          tunnel: w105 -> [w384]
          n199 = Negate(x=w394) -> (-x=w386:dbl)
          n200 = Negate(x=w392) -> (-x=w385:dbl)
          n201 = To Fixed-Point(fixed-point type=w384, number=w386) -> (fixed-point=w393:fxp<+/-,64,9>)
          n202 = To Fixed-Point(fixed-point type=w384, number=w385) -> (fixed-point=w389:fxp<+/-,64,9>)
          n203 = To Fixed-Point(fixed-point type=w384, number=w391) -> (fixed-point=w388:fxp<+/-,64,9>)
          n204 = To Fixed-Point(fixed-point type=w384, number=w390) -> (fixed-point=w387:fxp<+/-,64,9>)
        }
        "-a01(2) yz1c" <- w132
        "-a02(2) yz1c" <- w131
        "b01(2) yz1c" <- w130
        "b02(2) yz1c" <- w129
        n205 = for {
          tunnel: w287 -> [w496] mode=indexing
          tunnel: [w495] -> w293 mode=indexing
          tunnel: w286 -> [w494] mode=indexing
          tunnel: w289 -> [w493] mode=indexing
          tunnel: w288 -> [w492] mode=indexing
          tunnel: [w491] -> w292 mode=indexing
          tunnel: [w490] -> w291 mode=indexing
          tunnel: [w489] -> w290 mode=indexing
          tunnel: w105 -> [w486]
          n206 = Negate(x=w496) -> (-x=w488:dbl)
          n207 = Negate(x=w494) -> (-x=w487:dbl)
          n208 = To Fixed-Point(fixed-point type=w486, number=w488) -> (fixed-point=w495:fxp<+/-,64,9>)
          n209 = To Fixed-Point(fixed-point type=w486, number=w487) -> (fixed-point=w491:fxp<+/-,64,9>)
          n210 = To Fixed-Point(fixed-point type=w486, number=w493) -> (fixed-point=w490:fxp<+/-,64,9>)
          n211 = To Fixed-Point(fixed-point type=w486, number=w492) -> (fixed-point=w489:fxp<+/-,64,9>)
        }
        "-a01(2) zz1c" <- w293
        "-a02(2) zz1c" <- w292
        "b01(2) zz1c" <- w291
        "b02(2) zz1c" <- w290
        n212 = Divide(x=w363, y=1000) -> (x/y=→"Measured Controller Loop Rate (kHz)":dbl)
        n213 = Divide(x=w359, y=1000) -> (x/y=→"Measured Controller Output Loop Rate (kHz)":dbl)
        n214 = Divide(x=w355, y=1000) -> (x/y=→"Measured Plant Output Loop Rate (kHz)":dbl)
        n215 = Divide(x=w87, y=1000) -> (x/y=→"Measured Analog Input Loop Rate (kHz)":dbl)
      }
      frame "Update Reference Info" {
        w608 = 40000000.0  # FPGA Clock Rate (Hz)
        w602 = 1
        w615 = 40000000.0  # FPGA Clock Rate (Hz)
        w609 = 1
        w620 = errorcluster {"status"=FALSE, "code"=0, "source"=""}  # error in (no error)
        w623 = errorcluster {"status"=FALSE, "code"=0, "source"=""}  # error in (no error)
        w637 = 40000000.0  # FPGA Clock Rate (Hz)
        w631 = 1
        w649 = errorcluster {"status"=FALSE, "code"=0, "source"=""}  # error in (no error)
        w616 = 40000000.0  # FPGA clock rate (Hz)
        n216 = case shown="\"FPGA Snake Scan\", Default" "Snake Scan Reference FPGA or EPICS" {
          tunnel: ["X Ramp Start (nm)" w669] -> w544
          tunnel: ["X Ramp End (nm)" w668] -> w543
          tunnel: ["Fly Scan Start" w667] -> w542
          tunnel: ["Y Ramp Start (nm)" w666] -> w541
          tunnel: ["Y Ramp End (nm)" w665] -> w540
          tunnel: ["Y Vertical Step Size (nm)" w664] -> w539
          tunnel: ["X Horizontal Step Size (nm)" w663] -> w538
          tunnel: [w653 w661] -> w537
          frame "FPGA Snake Scan", Default {
            n217 = local read "DT Frequency (Hz)"() -> (w653:dbl)
          }
          frame "EPICS Snake Scan" {
            w662 = fxp<+/-,16,16> 0.0 ("fixed-point type")
            n218 = shared-variable "RT CompactRIO Target\\RT_EPICS_Shared_Variables.lvlib\\2iddVELO:Trigger_Freq_Hz"() -> (w661:dbl)  [unwired: 1 in, 1 out]
            n219 = shared-variable "RT CompactRIO Target\\RT_EPICS_Shared_Variables.lvlib\\2iddVELO:Y_Step_Size_nm"() -> (w671:dbl)  [unwired: 1 in, 1 out]
            n220 = shared-variable "RT CompactRIO Target\\RT_EPICS_Shared_Variables.lvlib\\2iddVELO:X_Step_Size_nm"() -> (w670:dbl)  [unwired: 1 in, 1 out]